vi "Host_sgl.vi"() -> ()   [LabVIEW 2019]
uses:
  <vilib>/Analysis/7linalg.llb/Eigenvalue and Vectors Output Option.ctl
  <vilib>/Analysis/baseanly.llb/Matrix Type of Inverse Matrix.ctl
  <vilib>/Analysis/7linalg.llb/Real Generalized Eigenvalues and Vectors.vi
  <vilib>/Analysis/7linalg.llb/Real Cholesky Factorization.vi
  <vilib>/Analysis/baseanly.llb/Full Cholesky Factorization.vi
  <vilib>/Analysis/baseanly.llb/Full Real Matrix Cholesky Factorization.vi
  <vilib>/FPGAPlugInAG/PXIe-7915/niLvFpga_Open_PXIe-7915.vi
  <vilib>/rvi/interface/common/dynamic/niFpgaDynamicAddResources.vi
  <vilib>/Analysis/baseanly.llb/Real Inverse Matrix.vi
  <vilib>/Analysis/Matrix/Numeric/Multiply/Multiply - RM,RM.vi
  <vilib>/Analysis/7linalg.llb/Real Eigenvalues and Vectors.vi
  <vilib>/Analysis/Matrix/Numeric/Add/Add - RM,RM.vi
  <vilib>/Utility/error.llb/Error Cluster From Error Code.vi
  <vilib>/rvi/errors/niLvFpgaAdjustHostInterfaceError.vi
  <vilib>/FPGAPlugInAG/Dynamic/niLvFpga_Run_Dynamic.vi
  <vilib>/FPGAPlugInAG/Dynamic/niLvFpga_Close_Dynamic.vi
  <vilib>/rvi/interface/nirviOpenFPGA/nirviOpenFPGA.xnode
  FPGA Bitfiles/choleskyfpgav1_FPGATarget_Target_xjOD3-+swO0.lvbitx
  Target.vi
  <vilib>/rvi/interface/nirviMethod/nirviMethod.xnode
  <vilib>/rvi/interface/nirviReadWriteControl/nirviReadWriteControl.xnode
  <vilib>/rvi/interface/nirviCloseFPGA/nirviCloseFPGA.xnode
  <vilib>/Analysis/NI_AALPro.lvlib
  <vilib>/Analysis/NI_AALBase.lvlib
  <vilib>/Analysis/Matrix/NI_Matrix.lvlib
  <vilib>/rvi/errors/niLvFpgaMergeErrorWithErrorCode.vi
  <vilib>/FPGAPlugInAG/Dynamic/niLvFpga_ReadFifo_Dynamic.vi
  <vilib>/FPGAPlugInAG/Dynamic/niLvFpga_WriteFifo_Dynamic.vi
  NiFpgaLv.dll
  <vilib>/rvi/interface/Simulation/niFpgaSimulationCallBeginRW.vi
panel:
  out "upload time":u32
  out "run time":u32
  out "load time":u32
  out "Elements Remaining 2":u32
  out "Elements Remaining":u32
  out "Frequencies":dbl[](array[numeric])
  out "Eigenvalues":cdb[][](array[numeric]) format="%#_4g"
  out "Boolean":bool
  out "K input":dbl[][](array[numeric])
  out "Run Time (ms)":u32 format="%_6f"
  in  "Method":i32(listbox)
  out "M input":dbl[][](array[numeric])
  # "Takes 56 ms to solve without timed loop"
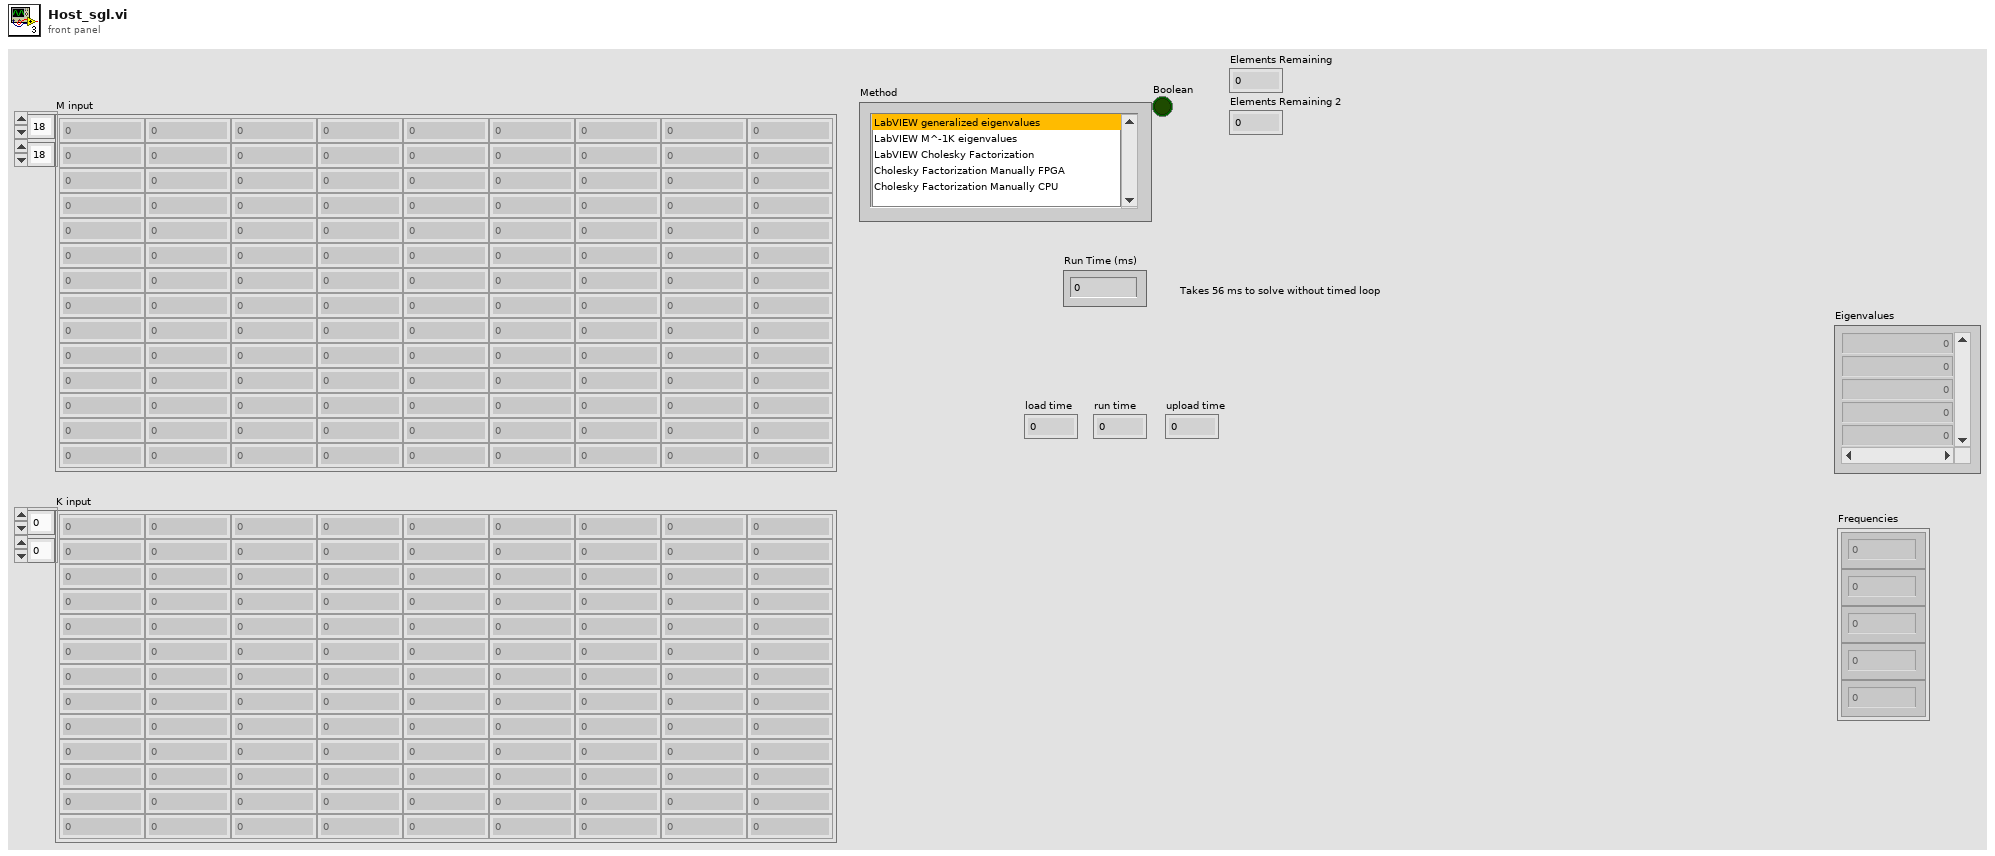
[diagram p1: front panel]
types:
  T1 = typedef "NI_AALBase.lvlib/Matrix Type of Inverse Matrix.ctl" = enum32{"General", "Positive Definite", "Lower Triangular", "Upper Triangular"}
  T2 = typedef "NI_AALPro.lvlib/Eigenvalue and Vectors Output Option.ctl" = i32
  T3 = typedef "NI_Matrix.lvlib/RealMatrix.ctl" = dbl[][]
  T4 = typedef "NI_Matrix.lvlib/ComplexMatrix.ctl" = cdb[][]
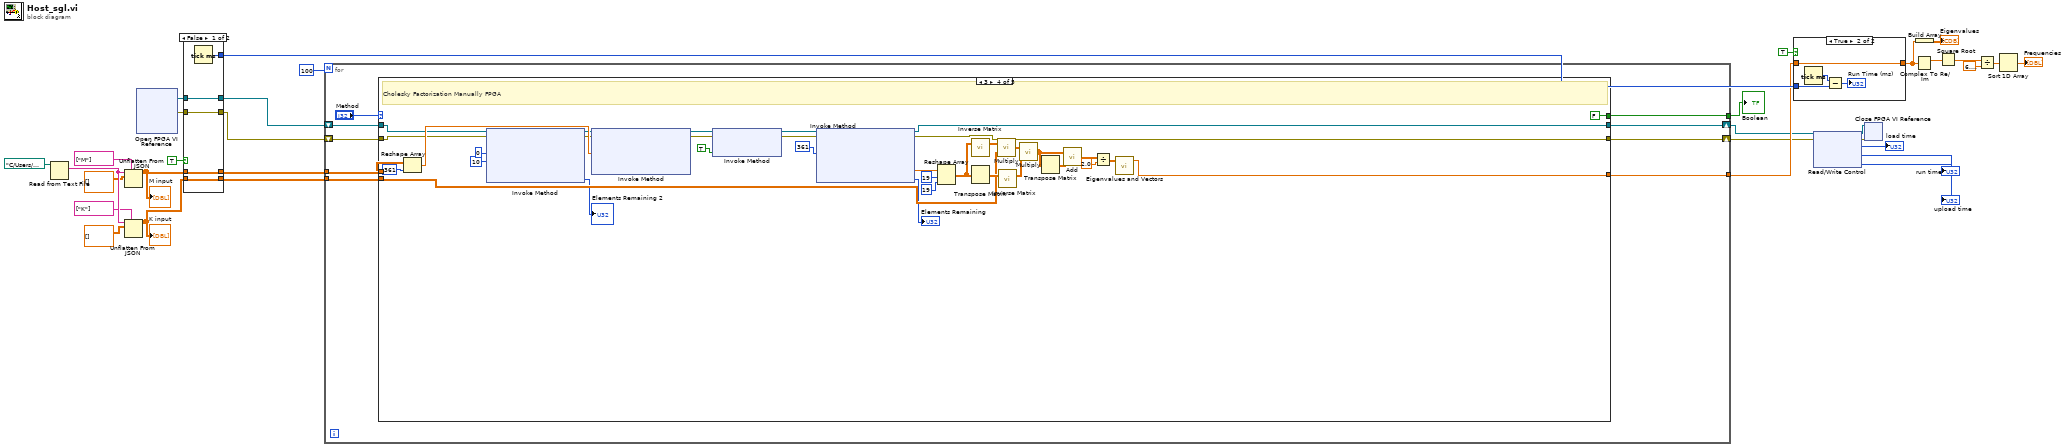
[diagram p0: block diagram]
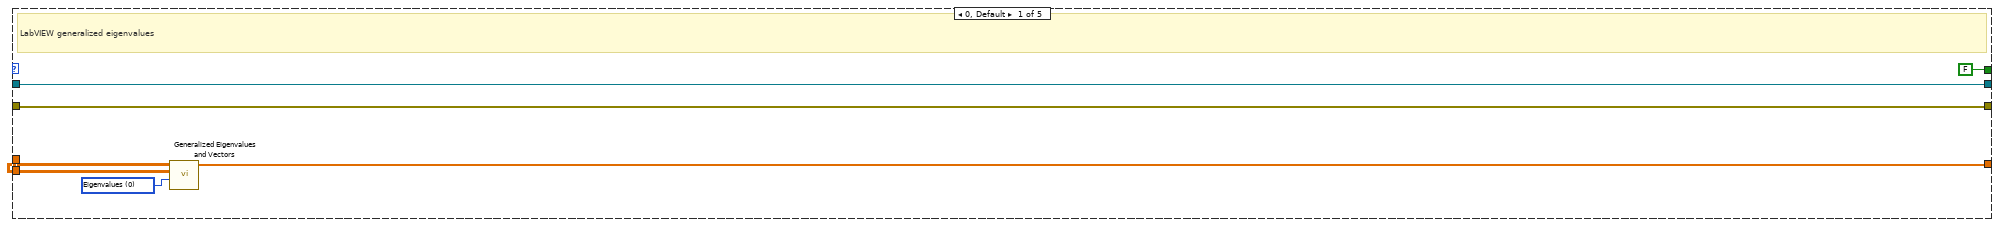
[diagram p2: hidden frame]
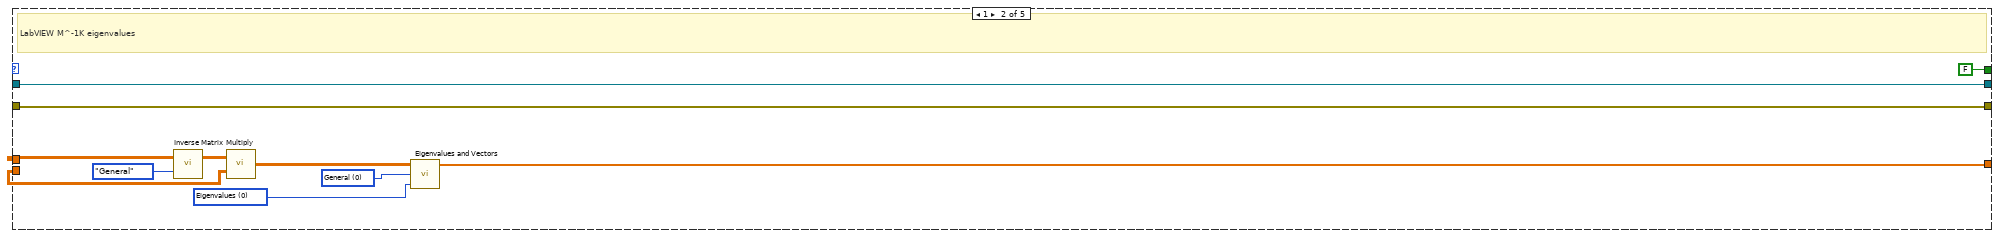
[diagram p3: hidden frame]
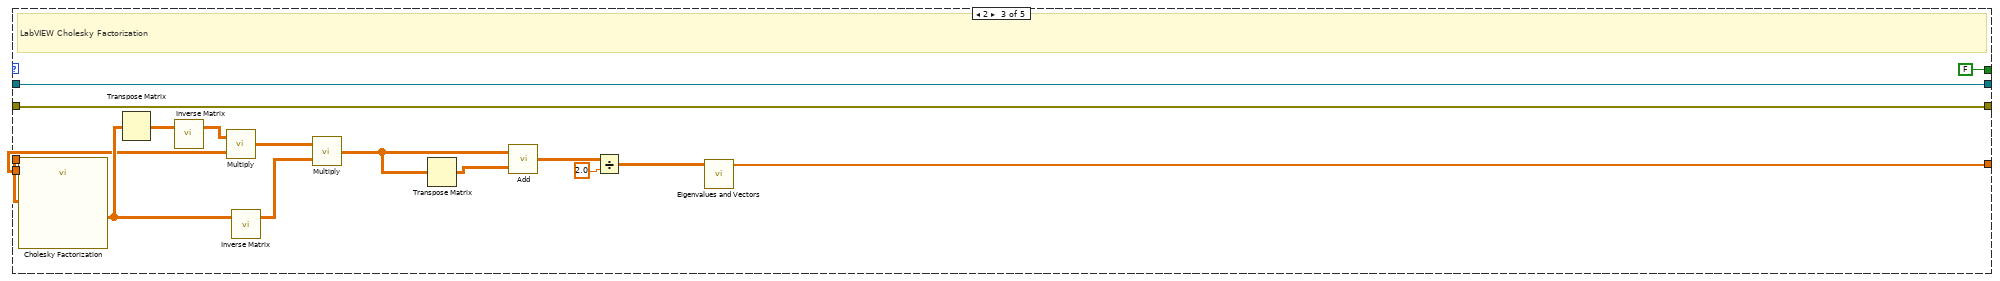
[diagram p4: hidden frame]
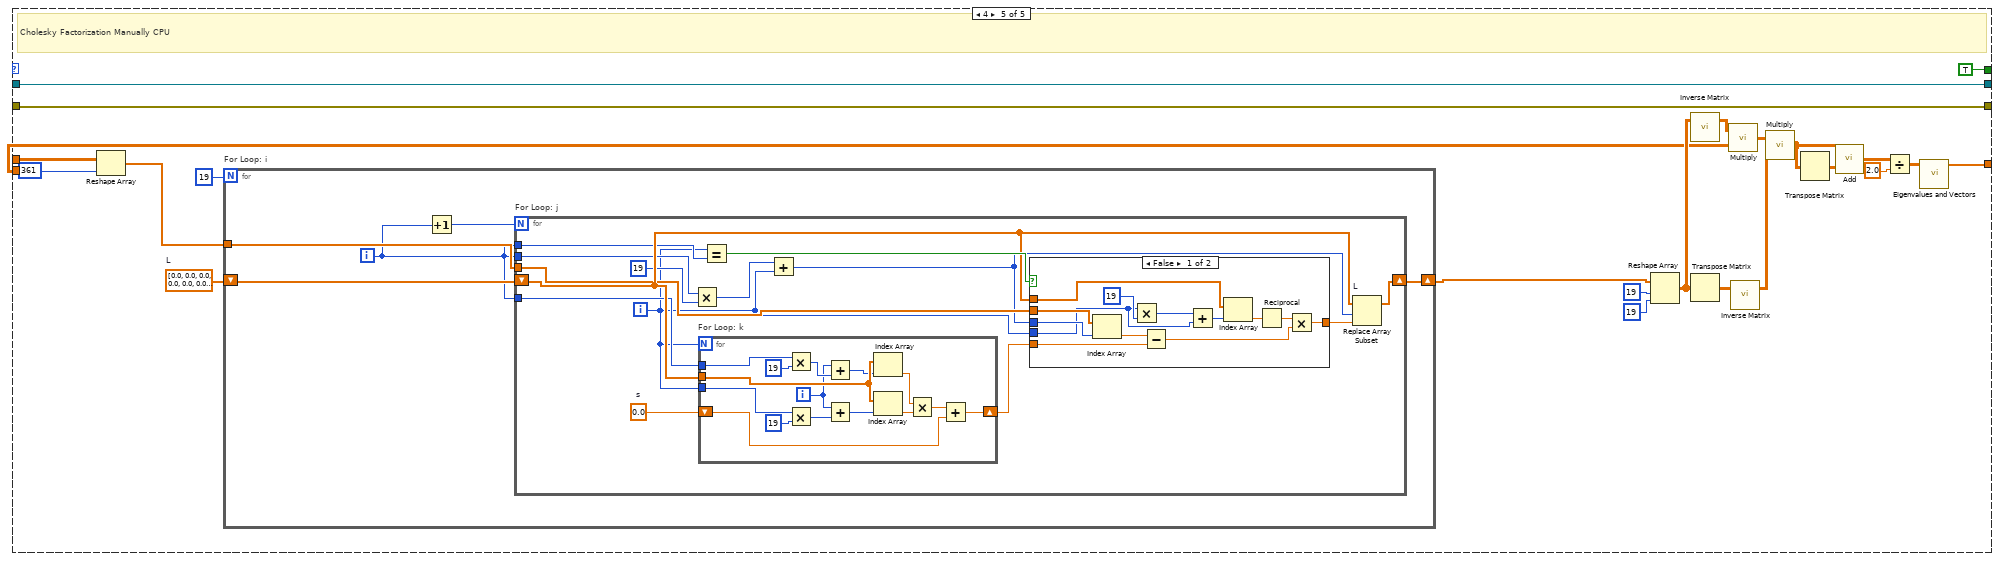
[diagram p5: hidden frame]
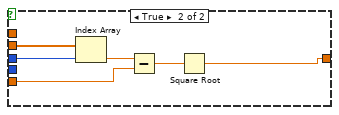
[diagram p6: hidden frame]
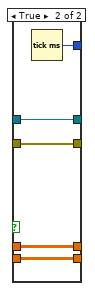
[diagram p8: hidden frame]
diagram:
  n1 = Read from Text File(file (use dialog)=path "C:/Users/PXIe-8880/Documents/AFRL_summer_2019/Cholesky_FPGA/Cholesky_FPGA_V1/data/data.txt") -> (text=w32:string)  [unwired: 3 in, 3 out]
  n2 = Unflatten From JSON(path=string[] ["M"], JSON string=w32, type and defaults=dbl[][] []) -> (value=w33:dbl[][])  [unwired: 4 in, 1 out]
  "M input" <- w33
  n3 = Unflatten From JSON(path=string[] ["K"], JSON string=w32, type and defaults=dbl[][] []) -> (value=w34:dbl[][])  [unwired: 4 in, 1 out]
  "K input" <- w34
  n4 = xnode "Open FPGA VI Reference"() -> ("FPGA VI Reference Out"=w12:refnum<k20>, "error out"=w10:errorcluster)  [unwired: 2 in]
  n5 = case shown="False" TRUE {
    tunnel: w33 -> [w39 w44]
    tunnel: [w39 w44] -> w25
    tunnel: w34 -> [w38 w43]
    tunnel: [w38 w43] -> w24
    tunnel: [w37 w42] -> w22
    tunnel: w12 -> [w36 w41]
    tunnel: [w36 w41] -> w11
    tunnel: w10 -> [w35 w40]
    tunnel: [w35 w40] -> w9
    frame False {
      n6 = Tick Count (ms)() -> (millisecond timer value=w37:u32)
    }
    frame True {
      n7 = Tick Count (ms)() -> (millisecond timer value=w42:u32)
    }
  }
  n8 = for {
    N: 100 -> [_]
    tunnel: w25 -> [w53]
    tunnel: w24 -> [w52]
    tunnel: [w49] -> w21
    tunnel: [w48] -> w13
    shift-right: [w51] -> w7
    shift-left: w11 -> [w46]
    shift-right: [w50] -> w6
    shift-left: w9 -> [w45]
    n9 = case shown="3" "Method" {
      tunnel: [w59 w67 w81 w106 w123] -> w48
      tunnel: w53 -> [w58 w66 w87 w122 w124]
      tunnel: w52 -> [w57 w65 w83 w107 w125]
      tunnel: w46 -> [w56 w63 w74 w93 w144]
      tunnel: [w56 w63 w74 w98 w144] -> w51
      tunnel: w45 -> [w55 w62 w73 w92 w143]
      tunnel: [w55 w62 w73 w99 w143] -> w50
      tunnel: [FALSE FALSE FALSE FALSE TRUE] -> w49
      frame 0, Default {
        w60 = T2 0 items=["Eigenvalues", "Eigenvalues & Vectors"] ("output option")
        # "LabVIEW generalized eigenvalues"
        n10 = call-poly <vilib>:"Generalized Eigenvalues and Vectors.vi"("output option"=w60, "B"=w58, "A"=w57) -> ("Eigenvalues"=w59:cdb[])  [unwired: 3 in, 2 out]
      }
      frame 1 {
        w68 = T2 0 items=["Eigenvalues", "Eigenvalues & Vectors"] ("output option")
        w69 = 0 items=["General", "Symmetric"] ("matrix type")
        # "LabVIEW M^-1K eigenvalues"
        n11 = call-poly <vilib>:"Inverse Matrix.vi"("matrix type"=Matrix_Type_of_Inverse_Matrix."General", "Input Matrix"=w66) -> ("Inverse Matrix"=w70:T3)  [unwired: 1 out]
        n12 = call-poly <vilib>:"Multiply.vi"("Real Matrix B"=w65, "Real Matrix A"=w70) -> ("A * B"=w71:T3)
        n13 = call-poly <vilib>:"Eigenvalues and Vectors.vi"("output option"=w68, "matrix type"=w69, "Input Matrix"=w71) -> ("Eigenvalues"=w67:cdb[])  [unwired: 2 out]
      }
      frame 2 {
        # "LabVIEW Cholesky Factorization"
        n14 = call-poly <vilib>:"Cholesky Factorization.vi"("A"=w87) -> ("Cholesky"=w85:T3)  [unwired: 1 out]
        n15 = Transpose Matrix(1:w85) -> (0:w86:T3)
        n16 = call-poly <vilib>:"Inverse Matrix.vi"("Input Matrix"=w86) -> ("Inverse Matrix"=w84:T3)  [unwired: 1 in, 1 out]
        n17 = call-poly <vilib>:"Multiply.vi"("Real Matrix B"=w83, "Real Matrix A"=w84) -> ("A * B"=w80:T3)
        n18 = call-poly <vilib>:"Inverse Matrix.vi"("Input Matrix"=w85) -> ("Inverse Matrix"=w82:T3)  [unwired: 1 in, 1 out]
        n19 = call-poly <vilib>:"Multiply.vi"("Real Matrix B"=w82, "Real Matrix A"=w80) -> ("A * B"=w79:T3)
        n20 = Transpose Matrix(1:w79) -> (0:w78:T3)
        n21 = call-poly <vilib>:"Add.vi"("Real Matrix B"=w78, "Real Matrix A"=w79) -> ("A + B"=w76:T3)
        n22 = Divide(x=w76, y=2.0) -> (x/y=w75:T3)
        n23 = call-poly <vilib>:"Eigenvalues and Vectors.vi"("Input Matrix"=w75) -> ("Eigenvalues"=w81:cdb[])  [unwired: 2 in, 2 out]
      }
      frame 3 {
        # "Cholesky Factorization Manually FPGA"
        n24 = Reshape Array(w122, 361 ("dimension size")) -> (w102:dbl[])
        n25 = xnode "Invoke Method"("FPGA VI Reference In"=w93, "error in"=w92, "Number of Elements"=u32 0, "Timeout (ms)"=10) -> ("FPGA VI Reference Out"=w91:refnum<k20>, "error out"=w90:errorcluster, "Elements Remaining"=→"Elements Remaining 2":u32)  [unwired: 1 out]
        n26 = xnode "Invoke Method"("FPGA VI Reference In"=w91, "error in"=w90, "Data"=w102) -> ("FPGA VI Reference Out"=w104:refnum<k20>, "error out"=w103:errorcluster)  [unwired: 1 in, 1 out]
        n27 = xnode "Invoke Method"("FPGA VI Reference In"=w104, "error in"=w103, "Wait Until Done (F)"=TRUE) -> ("FPGA VI Reference Out"=w101:refnum<k20>, "error out"=w100:errorcluster)
        n28 = xnode "Invoke Method"("FPGA VI Reference In"=w101, "error in"=w100, "Number of Elements"=u32 361) -> ("FPGA VI Reference Out"=w98:refnum<k20>, "error out"=w99:errorcluster, "Data"=w96:sgl[], "Elements Remaining"=→"Elements Remaining":u32)  [unwired: 1 in]
        n29 = Reshape Array(w96, 19 ("dimension size"), 19 ("dimension size")) -> (w108:sgl[][])
        n30 = call-poly <vilib>:"Inverse Matrix.vi"("Input Matrix"=w108) -> ("Inverse Matrix"=w117:T3)  [unwired: 1 in, 1 out]
        n31 = Transpose Matrix(1:w108) -> (0:w109:dbl[][])
        n32 = call-poly <vilib>:"Multiply.vi"("Real Matrix B"=w107, "Real Matrix A"=w117) -> ("A * B"=w115:T3)
        n33 = call-poly <vilib>:"Inverse Matrix.vi"("Input Matrix"=w109) -> ("Inverse Matrix"=w116:T3)  [unwired: 1 in, 1 out]
        n34 = call-poly <vilib>:"Multiply.vi"("Real Matrix B"=w116, "Real Matrix A"=w115) -> ("A * B"=w114:T3)
        n35 = Transpose Matrix(1:w114) -> (0:w113:T3)
        n36 = call-poly <vilib>:"Add.vi"("Real Matrix B"=w113, "Real Matrix A"=w114) -> ("A + B"=w111:T3)
        n37 = Divide(x=w111, y=2.0) -> (x/y=w110:T3)
        n38 = call-poly <vilib>:"Eigenvalues and Vectors.vi"("Input Matrix"=w110) -> ("Eigenvalues"=w106:cdb[])  [unwired: 2 in, 2 out]
      }
      frame 4 {
        w142 = sgl[] [0.0, 0.0, 0.0, 0.0, 0.0, 0.0, 0.0, 0.0, 0.0, 0.0, 0.0, 0.0, 0.0, 0.0, 0.0, 0.0, 0.0, 0.0, 0.0, 0.0, 0.0, 0.0, 0.0, 0.0, 0.0, 0.0, 0.0, 0.0, 0.0, 0.0, 0.0, 0.0, 0.0, 0.0, 0.0, 0.0, 0.0, 0.0, 0.0, 0.0, 0.0, 0.0, 0.0, 0.0, 0.0, 0.0, 0.0, 0.0, 0.0, 0.0, 0.0, 0.0, 0.0, 0.0, 0.0, 0.0, 0.0, 0.0, 0.0, 0.0, 0.0, 0.0, 0.0, 0.0, 0.0, 0.0, 0.0, 0.0, 0.0, 0.0, 0.0, 0.0, 0.0, 0.0, 0.0, 0.0, 0.0, 0.0, 0.0, 0.0, 0.0, 0.0, 0.0, 0.0, 0.0, 0.0, 0.0, 0.0, 0.0, 0.0, 0.0, 0.0, 0.0, 0.0, 0.0, 0.0, 0.0, 0.0, 0.0, 0.0, 0.0, 0.0, 0.0, 0.0, 0.0, 0.0, 0.0, 0.0, 0.0, 0.0, 0.0, 0.0, 0.0, 0.0, 0.0, 0.0, 0.0, 0.0, 0.0, 0.0, 0.0, 0.0, 0.0, 0.0, 0.0, 0.0, 0.0, 0.0, 0.0, 0.0, 0.0, 0.0, 0.0, 0.0, 0.0, 0.0, 0.0, 0.0, 0.0, 0.0, 0.0, 0.0, 0.0, 0.0, 0.0, 0.0, 0.0, 0.0, 0.0, 0.0, 0.0, 0.0, 0.0, 0.0, 0.0, 0.0, 0.0, 0.0, 0.0, 0.0, 0.0, 0.0, 0.0, 0.0, 0.0, 0.0, 0.0, 0.0, 0.0, 0.0, 0.0, 0.0, 0.0, 0.0, 0.0, 0.0, 0.0, 0.0, 0.0, 0.0, 0.0, 0.0, 0.0, 0.0, 0.0, 0.0, 0.0, 0.0, 0.0, 0.0, 0.0, 0.0, 0.0, 0.0, 0.0, 0.0, 0.0, 0.0, 0.0, 0.0, 0.0, 0.0, 0.0, 0.0, 0.0, 0.0, 0.0, 0.0, 0.0, 0.0, 0.0, 0.0, 0.0, 0.0, 0.0, 0.0, 0.0, 0.0, 0.0, 0.0, 0.0, 0.0, 0.0, 0.0, 0.0, 0.0, 0.0, 0.0, 0.0, 0.0, 0.0, 0.0, 0.0, 0.0, 0.0, 0.0, 0.0, 0.0, 0.0, 0.0, 0.0, 0.0, 0.0, 0.0, 0.0, 0.0, 0.0, 0.0, 0.0, 0.0, 0.0, 0.0, 0.0, 0.0, 0.0, 0.0, 0.0, 0.0, 0.0, 0.0, 0.0, 0.0, 0.0, 0.0, 0.0, 0.0, 0.0, 0.0, 0.0, 0.0, 0.0, 0.0, 0.0, 0.0, 0.0, 0.0, 0.0, 0.0, 0.0, 0.0, 0.0, 0.0, 0.0, 0.0, 0.0, 0.0, 0.0, 0.0, 0.0, 0.0, 0.0, 0.0, 0.0, 0.0, 0.0, 0.0, 0.0, 0.0, 0.0, 0.0, 0.0, 0.0, 0.0, 0.0, 0.0, 0.0, 0.0, 0.0, 0.0, 0.0, 0.0, 0.0, 0.0, 0.0, 0.0, 0.0, 0.0, 0.0, 0.0, 0.0, 0.0, 0.0, 0.0, 0.0, 0.0, 0.0, 0.0, 0.0, 0.0, 0.0, 0.0, 0.0, 0.0, 0.0, 0.0, 0.0, 0.0, 0.0, 0.0, 0.0, 0.0, 0.0, 0.0, 0.0, 0.0, 0.0, 0.0, 0.0, 0.0, 0.0, 0.0, 0.0, 0.0, 0.0, 0.0, 0.0, 0.0, 0.0, 0.0, 0.0, 0.0]  # L
        # "Cholesky Factorization Manually CPU"
        n39 = Reshape Array(w124, 361 ("dimension size")) -> (w139:dbl[])
        n40 = for "For Loop: i" {
          N: 19 -> [_]
          shift-right: [w148] -> w127
          shift-left: w142 -> [w150]
          tunnel: w139 -> [w147]
          i -> [w146]
          n41 = Increment(x=w146) -> (x+1=w149:i32)
          n42 = for "For Loop: j" {
            N: w149 -> [_]
            tunnel: w146 -> [w158]
            shift-right: [w160] -> w148
            shift-left: w150 -> [w159]
            tunnel: w146 -> [w157]
            tunnel: w147 -> [w154]
            tunnel: w146 -> [w152]
            i -> [w151]
            w163 = sgl 0.0  # s
            n43 = Multiply(x=w157, y=19) -> (x*y=w155:i32)
            n44 = for "For Loop: k" {
              N: w151 -> [_]
              tunnel: w159 -> [w197]
              shift-right: [w193] -> w162
              shift-left: w163 -> [w194]
              tunnel: w152 -> [w192]
              tunnel: w151 -> [w185]
              i -> [w184]
              n45 = Multiply(x=w192, y=19) -> (x*y=w190:i32)
              n46 = Multiply(x=w185, y=19) -> (x*y=w187:i32)
              n47 = Add(x=w184, y=w190) -> (x+y=w189:i32)
              n48 = Add(x=w184, y=w187) -> (x+y=w186:i32)
              n49 = Index Array(array=w197, index=w189) -> (element=w198:sgl)
              n50 = Index Array(array=w197, index=w186) -> (element=w196:sgl)
              n51 = Multiply(x=w198, y=w196) -> (x*y=w195:sgl)
              n52 = Add(x=w195, y=w194) -> (x+y=w193:sgl)
            }
            n53 = Equal?(x=w151, y=w158) -> (x = y?=w164:bool)
            n54 = Add(x=w155, y=w151) -> (x+y=w153:i32)
            n55 = case shown="False" w164 {
              tunnel: w162 -> [w175 w183]
              tunnel: [w174 w181] -> w161
              tunnel: w159 -> [w177 _]
              tunnel: w154 -> [w171 w180]
              tunnel: w153 -> [w170 w179]
              tunnel: w151 -> [w166 _]
              frame False {
                n56 = Index Array(array=w171, index=w170) -> (element=w169:dbl)
                n57 = Multiply(x=w166, y=19) -> (x*y=w167:i32)
                n58 = Subtract(x=w169, y=w175) -> (x-y=w172:dbl)
                n59 = Add(x=w167, y=w166) -> (x+y=w165:i32)
                n60 = Index Array(array=w177, index=w165) -> (element=w176:sgl)
                n61 = Reciprocal(x=w176) -> (1/x=w173:sgl)
                n62 = Multiply(x=w173, y=w172) -> (x*y=w174:dbl)
              }
              frame True {
                n63 = Index Array(array=w180, index=w179) -> (element=w178:dbl)
                n64 = Subtract(x=w178, y=w183) -> (x-y=w182:dbl)
                n65 = Square Root(x=w182) -> (sqrt(x)=w181:dbl)
              }
            }
            n66 = Replace Array Subset "L"(array=w159, new element=w161, index=w153) -> (w160:sgl[])
          }
        }
        n67 = Reshape Array(w127, 19 ("dimension size"), 19 ("dimension size")) -> (w126:sgl[][])
        n68 = call-poly <vilib>:"Inverse Matrix.vi"("Input Matrix"=w126) -> ("Inverse Matrix"=w136:T3)  [unwired: 1 in, 1 out]
        n69 = Transpose Matrix(1:w126) -> (0:w128:dbl[][])
        n70 = call-poly <vilib>:"Multiply.vi"("Real Matrix B"=w125, "Real Matrix A"=w136) -> ("A * B"=w134:T3)
        n71 = call-poly <vilib>:"Inverse Matrix.vi"("Input Matrix"=w128) -> ("Inverse Matrix"=w135:T3)  [unwired: 1 in, 1 out]
        n72 = call-poly <vilib>:"Multiply.vi"("Real Matrix B"=w135, "Real Matrix A"=w134) -> ("A * B"=w133:T3)
        n73 = Transpose Matrix(1:w133) -> (0:w132:T3)
        n74 = call-poly <vilib>:"Add.vi"("Real Matrix B"=w132, "Real Matrix A"=w133) -> ("A + B"=w130:T3)
        n75 = Divide(x=w130, y=2.0) -> (x/y=w129:T3)
        n76 = call-poly <vilib>:"Eigenvalues and Vectors.vi"("Input Matrix"=w129) -> ("Eigenvalues"=w123:cdb[])  [unwired: 2 in, 2 out]
      }
    }
  }
  "Boolean" <- w21
  n77 = case shown="True" TRUE {
    tunnel: w22 -> [_ w202]
    tunnel: [w199 w200] -> w14
    tunnel: w13 -> [w199 w200]
    frame False {
    }
    frame True {
      n78 = Tick Count (ms)() -> (millisecond timer value=w203:u32)
      n79 = Subtract(x=w203, y=w202) -> (x-y=→"Run Time (ms)":u32)
    }
  }
  n80 = xnode "Read/Write Control"("FPGA VI Reference In"=w7, "error in"=w6) -> ("FPGA VI Reference Out"=w5:refnum<k20>, "error out"=w4:errorcluster, "load time"=→"load time":u32, "run time"=→"run time":u32, "upload time"=→"upload time":u32)
  n81 = xnode "Close FPGA VI Reference"("FPGA VI Reference In"=w5, "error in"=w4) -> ()  [unwired: 1 out]
  n82 = Build Array(w14) -> (→"Eigenvalues":T4)
  n83 = Complex To Re/Im ("Complex To Cartesian.vi")(x + iy=w14) -> (x=w18:dbl[])  [unwired: 1 out]
  n84 = Square Root ("Square Root.vi")(x=w18) -> (sqrt(x)=w19:dbl[])
  n85 = Divide(x=w19, y=6.283185307179586) -> (x/y=w20:dbl[])
  n86 = Sort 1D Array(array=w20) -> (sorted array=→"Frequencies":dbl[])
